vi "TLB Native Dynamic Events ver 0.26a.vi"() -> ()   [LabVIEW 2018] (continued)
              tunnel: [w1090 State_Type_Definitions,_for_0.26g_versions_and_later_2."True Stop" ("Enum")] -> w1083
              tunnel: [w1093 w1110] -> w1076
              tunnel: [State_Type_Definitions,_for_0.26g_versions_and_later_2."Idle" ("Enum") State_Type_Definitions,_for_0.26g_versions_and_later_2."Shutdown" ("Enum")] -> w1075
              tunnel: w1077 -> [w1084 _]
              tunnel: w1082 -> [w1089 w1107]
              tunnel: w1069 -> [w1088 _]
              frame "Start Task 1", Default {
                # ">> Is time up? >>"
                # "Determines if object is in range to pick up"
                # ">> Manual override >>"
                n408 = case shown="True" w1088 {
                  tunnel: [w1097 w1103] -> w1093
                  tunnel: w1089 -> [w1095 w1101]
                  frame False {
                    n409 = for {
                      tunnel: string[] ["Z STEPPER CAM HEIGHT", "READ STEPPER VALUES"] ("element") -> [w1098] mode=indexing
                      shift-right: [w1100] -> w1097
                      shift-left: w1095 -> [w1099]
                      n410 = Enqueue Element(queue=w1099, element=w1098) -> (queue out=w1100:refnum<queue>)  [unwired: 2 in, 2 out]
                    }
                  }
                  frame True {
                    n411 = for {
                      shift-right: [w1105] -> w1103
                      shift-left: w1101 -> [w1106]
                      tunnel: string[] ["SET TIMER 5", "", ""] -> [w1104] mode=indexing
                      n412 = Enqueue Element(queue=w1106, element=w1104) -> (queue out=w1105:refnum<queue>)  [unwired: 2 in, 2 out]
                    }
                  }
                }
                n413 = Or(x=w1088, y=w1084) -> (x .or. y?=w1091:bool)
                n414 = Select(t=State_Type_Definitions,_for_0.26g_versions_and_later_2."True Stop" ("Enum"), s=w1084, f=State_Type_Definitions,_for_0.26g_versions_and_later_2."Task 5D" ("Enum")) -> (s? t:f=w1086:T18)
                n415 = Select(t=w1086, s=w1091, f=State_Type_Definitions,_for_0.26g_versions_and_later_2."Task 5C" ("Enum")) -> (s? t:f=w1090:T18)
              }
              frame "Exit" {
                n416 = for {
                  shift-right: [w1113] -> w1110
                  shift-left: w1107 -> [w1114]
                  tunnel: string[] ["STOP", "RESET ENCODERS", "RESET YAW", "ARDUINO MODE 0"] -> [w1112] mode=indexing
                  n417 = Enqueue Element(queue=w1114, element=w1112) -> (queue out=w1113:refnum<queue>)  [unwired: 2 in, 2 out]
                }
              }
            }
          }
          frame 19 {
            # ">>> yStepper command>>>"
            n418 = Dequeue Element(queue=w1122, timeout in ms (-1)=w1121, error in (no error)=w1120) -> (element=w1119:T10)  [unwired: 3 out]
            n419 = case shown="\"Start Task 1\", Default" w1119 {
              tunnel: [w1134 State_Type_Definitions,_for_0.26g_versions_and_later_2."True Stop" ("Enum")] -> w1126
              tunnel: [w1137 w1154] -> w1125
              tunnel: [State_Type_Definitions,_for_0.26g_versions_and_later_2."Idle" ("Enum") State_Type_Definitions,_for_0.26g_versions_and_later_2."Shutdown" ("Enum")] -> w1127
              tunnel: w1123 -> [w1133 _]
              tunnel: w1124 -> [w1129 w1151]
              tunnel: w1117 -> [w1128 _]
              frame "Start Task 1", Default {
                # ">> T: Breaks out of state loop; F: Stays in loop>>"
                # ">> Manual override >>"
                # ">> Checks if time is up>>"
                # "Stays in Task 5D until the object is detected"
                # "T: Go back to idle, F: Continue with task\""
                # ">> Manual override >>"
                n420 = case shown="False" w1128 {
                  tunnel: [w1141 w1147] -> w1137
                  tunnel: w1129 -> [w1139 w1145]
                  frame False {
                    n421 = for {
                      tunnel: string[] ["START TIMER", "OPEN CLAW", ""] ("element") -> [w1142] mode=indexing
                      shift-right: [w1144] -> w1141
                      shift-left: w1139 -> [w1143]
                      n422 = Enqueue Element(queue=w1143, element=w1142) -> (queue out=w1144:refnum<queue>)  [unwired: 2 in, 2 out]
                    }
                  }
                  frame True {
                    n423 = for {
                      shift-right: [w1149] -> w1147
                      shift-left: w1145 -> [w1150]
                      tunnel: string[] ["CAM CLOSE", "", ""] -> [w1148] mode=indexing
                      n424 = Enqueue Element(queue=w1150, element=w1148) -> (queue out=w1149:refnum<queue>)  [unwired: 2 in, 2 out]
                    }
                  }
                }
                n425 = Or(x=w1128, y=w1133) -> (x .or. y?=w1135:bool)
                n426 = Select(t=State_Type_Definitions,_for_0.26g_versions_and_later_2."True Stop" ("Enum"), s=w1133, f=State_Type_Definitions,_for_0.26g_versions_and_later_2."True Stop" ("Enum")) -> (s? t:f=w1130:T18)
                n427 = Select(t=w1130, s=w1135, f=State_Type_Definitions,_for_0.26g_versions_and_later_2."Task 5D" ("Enum")) -> (s? t:f=w1134:T18)
              }
              frame "Exit" {
                n428 = for {
                  shift-right: [w1157] -> w1154
                  shift-left: w1151 -> [w1158]
                  tunnel: string[] ["STOP", "RESET ENCODERS", "RESET YAW", "ARDUINO MODE 0"] -> [w1156] mode=indexing
                  n429 = Enqueue Element(queue=w1158, element=w1156) -> (queue out=w1157:refnum<queue>)  [unwired: 2 in, 2 out]
                }
              }
            }
          }
          frame 20 {
            # ">>> yStepper command>>>"
            n430 = Dequeue Element(queue=w1172, timeout in ms (-1)=w1173, error in (no error)=w1174) -> (element=w1176:T10)  [unwired: 3 out]
            n431 = formula code="if (pos < 100)\ny = 41;\n\nelse if (pos >= 100 && pos <= 140)\ny = 30;\n\nelse if (pos >= 141 && pos <= 170)\ny = 25;\n\nelse if (pos >= 171 &&pos <= 180) \ny = 20;\n\nelse if (pos >= 181&& pos <= 200)\ny = 15;\n\nelse if (pos >= 201 && pos <= 230)\ny = 10;\n\nelse if (pos >= 231 && pos <= 320)\ny = 8;\n\nelse if (pos > 320)\ny = 0;"("pos"=w1164) -> ("y"=w1167:dbl)
            n432 = To Unsigned Byte Integer(number=w1167) -> (unsigned 8bit integer=w1162:u8)
            n433 = Equal?(x=w1163, y=w1162) -> (x = y?=w1161:bool)
            n434 = case shown="\"Start Task 1\", Default" w1176 {
              tunnel: [w1183 State_Type_Definitions,_for_0.26g_versions_and_later_2."True Stop" ("Enum")] -> w1170
              tunnel: [w1186 w1203] -> w1168
              tunnel: [State_Type_Definitions,_for_0.26g_versions_and_later_2."Idle" ("Enum") State_Type_Definitions,_for_0.26g_versions_and_later_2."Shutdown" ("Enum")] -> w1169
              tunnel: w1175 -> [w1182 _]
              tunnel: w1171 -> [w1178 w1200]
              tunnel: w1161 -> [w1177 _]
              frame "Start Task 1", Default {
                # ">> T: Breaks out of state loop; F: Stays in loop>>"
                # ">> Manual override >>"
                # ">> Checks if time is up>>"
                # "Stays in Task 5D until the object is detected"
                # "T: Go back to idle, F: Continue with task\""
                # ">> Manual override >>"
                n435 = case shown="False" w1177 {
                  tunnel: [w1190 w1196] -> w1186
                  tunnel: w1178 -> [w1188 w1194]
                  frame False {
                    n436 = for {
                      tunnel: string[] ["READ STEPPER VALUES", "Y STEPPER CONTROL", ""] ("element") -> [w1191] mode=indexing
                      shift-right: [w1193] -> w1190
                      shift-left: w1188 -> [w1192]
                      n437 = Enqueue Element(queue=w1192, element=w1191) -> (queue out=w1193:refnum<queue>)  [unwired: 2 in, 2 out]
                    }
                  }
                  frame True {
                    n438 = for {
                      shift-right: [w1198] -> w1196
                      shift-left: w1194 -> [w1199]
                      tunnel: string[] ["CAM CLOSE", "DISPOSE BUFFERS", ""] -> [w1197] mode=indexing
                      n439 = Enqueue Element(queue=w1199, element=w1197) -> (queue out=w1198:refnum<queue>)  [unwired: 2 in, 2 out]
                    }
                  }
                }
                n440 = Or(x=w1177, y=w1182) -> (x .or. y?=w1184:bool)
                n441 = Select(t=State_Type_Definitions,_for_0.26g_versions_and_later_2."True Stop" ("Enum"), s=w1182, f=State_Type_Definitions,_for_0.26g_versions_and_later_2."Task 5F: ARM GRAB HEIGHT" ("Enum")) -> (s? t:f=w1179:T18)
                n442 = Select(t=w1179, s=w1184, f=State_Type_Definitions,_for_0.26g_versions_and_later_2."Task 5E: POSITION ARM" ("Enum")) -> (s? t:f=w1183:T18)
              }
              frame "Exit" {
                n443 = for {
                  shift-right: [w1206] -> w1203
                  shift-left: w1200 -> [w1207]
                  tunnel: string[] ["STOP", "RESET ENCODERS", "RESET YAW", "ARDUINO MODE 0"] -> [w1205] mode=indexing
                  n444 = Enqueue Element(queue=w1207, element=w1205) -> (queue out=w1206:refnum<queue>)  [unwired: 2 in, 2 out]
                }
              }
            }
            n445 = Bundle By Name(cluster=w1166, "yStepper desired"=w1162) -> (w1165:T20)
          }
          frame 21 {
            # ">>> Motor control cluster >>>"
            # ">>> yStepper command>>>"
            # ">> Manual override >>"
            n446 = Dequeue Element(queue=w1218, timeout in ms (-1)=w1217, error in (no error)=w1219) -> (element=w1216:T10)  [unwired: 3 out]
            n447 = Equal?(x=w1215, y=u8 1) -> (x = y?=w1213:bool)
            n448 = case shown="\"Start Task 1\", Default" w1216 {
              tunnel: [w1229 State_Type_Definitions,_for_0.26g_versions_and_later_2."True Stop" ("Enum")] -> w1220
              tunnel: [w1232 w1249] -> w1221
              tunnel: [State_Type_Definitions,_for_0.26g_versions_and_later_2."Idle" ("Enum") State_Type_Definitions,_for_0.26g_versions_and_later_2."Shutdown" ("Enum")] -> w1222
              tunnel: w1213 -> [w1228 _]
              tunnel: w1212 -> [w1227 _]
              tunnel: w1211 -> [w1223 w1246]
              frame "Start Task 1", Default {
                # "Stays in Task 5F until stepper reaches desired \nheight"
                # "T: Go back to idle, F: Continue with task\""
                # ">> Manual override >>"
                n449 = case shown="True" w1228 {
                  tunnel: [w1236 w1242] -> w1232
                  tunnel: w1223 -> [w1234 w1240]
                  frame False {
                    n450 = for {
                      tunnel: string[] ["Z STEPPER GRAB HEIGHT", "READ STEPPER VALUES"] ("element") -> [w1237] mode=indexing
                      shift-right: [w1239] -> w1236
                      shift-left: w1234 -> [w1238]
                      n451 = Enqueue Element(queue=w1238, element=w1237) -> (queue out=w1239:refnum<queue>)  [unwired: 2 in, 2 out]
                    }
                  }
                  frame True {
                    n452 = for {
                      shift-right: [w1244] -> w1242
                      shift-left: w1240 -> [w1245]
                      tunnel: string[] ["SET TIMER 5", "CLOSE CLAW", ""] -> [w1243] mode=indexing
                      n453 = Enqueue Element(queue=w1245, element=w1243) -> (queue out=w1244:refnum<queue>)  [unwired: 2 in, 2 out]
                    }
                  }
                }
                n454 = Or(x=w1228, y=w1227) -> (x .or. y?=w1230:bool)
                n455 = Select(t=State_Type_Definitions,_for_0.26g_versions_and_later_2."True Stop" ("Enum"), s=w1227, f=State_Type_Definitions,_for_0.26g_versions_and_later_2."Task 5G: CLOSE CLAW" ("Enum")) -> (s? t:f=w1224:T18)
                n456 = Select(t=w1224, s=w1230, f=State_Type_Definitions,_for_0.26g_versions_and_later_2."Task 5F: ARM GRAB HEIGHT" ("Enum")) -> (s? t:f=w1229:T18)
              }
              frame "Exit" {
                n457 = for {
                  shift-right: [w1252] -> w1249
                  shift-left: w1246 -> [w1253]
                  tunnel: string[] ["STOP", "RESET ENCODERS", "RESET YAW", "ARDUINO MODE 0"] -> [w1251] mode=indexing
                  n458 = Enqueue Element(queue=w1253, element=w1251) -> (queue out=w1252:refnum<queue>)  [unwired: 2 in, 2 out]
                }
              }
            }
          }
          frame 22 {
            # ">>> yStepper command>>>"
            # ">> Manual override >>"
            n459 = Dequeue Element(queue=w1264, timeout in ms (-1)=w1263, error in (no error)=w1262) -> (element=w1261:T10)  [unwired: 3 out]
            n460 = case shown="\"Start Task 1\", Default" w1261 {
              tunnel: [w1273 State_Type_Definitions,_for_0.26g_versions_and_later_2."True Stop" ("Enum")] -> w1266
              tunnel: [w1276 w1293] -> w1259
              tunnel: [State_Type_Definitions,_for_0.26g_versions_and_later_2."Idle" ("Enum") State_Type_Definitions,_for_0.26g_versions_and_later_2."Shutdown" ("Enum")] -> w1258
              tunnel: w1260 -> [w1267 _]
              tunnel: w1265 -> [w1272 w1290]
              tunnel: w1256 -> [w1271 _]
              frame "Start Task 1", Default {
                # ">> Is time up? >>"
                # "Determines if object is in range to pick up"
                # ">> Manual override >>"
                n461 = case shown="True" w1271 {
                  tunnel: [w1280 w1286] -> w1276
                  tunnel: w1272 -> [w1278 w1284]
                  frame False {
                    n462 = for {
                      tunnel: string[] ["CLOSE CLAW", "START TIMER"] ("element") -> [w1281] mode=indexing
                      shift-right: [w1283] -> w1280
                      shift-left: w1278 -> [w1282]
                      n463 = Enqueue Element(queue=w1282, element=w1281) -> (queue out=w1283:refnum<queue>)  [unwired: 2 in, 2 out]
                    }
                  }
                  frame True {
                    n464 = for {
                      shift-right: [w1288] -> w1286
                      shift-left: w1284 -> [w1289]
                      tunnel: string[] ["READ STEPPER VALUES", "", ""] -> [w1287] mode=indexing
                      n465 = Enqueue Element(queue=w1289, element=w1287) -> (queue out=w1288:refnum<queue>)  [unwired: 2 in, 2 out]
                    }
                  }
                }
                n466 = Or(x=w1271, y=w1267) -> (x .or. y?=w1274:bool)
                n467 = Select(t=State_Type_Definitions,_for_0.26g_versions_and_later_2."True Stop" ("Enum"), s=w1267, f=State_Type_Definitions,_for_0.26g_versions_and_later_2."Task 5H: RAISE ARM" ("Enum")) -> (s? t:f=w1269:T18)
                n468 = Select(t=w1269, s=w1274, f=State_Type_Definitions,_for_0.26g_versions_and_later_2."Task 5G: CLOSE CLAW" ("Enum")) -> (s? t:f=w1273:T18)
              }
              frame "Exit" {
                n469 = for {
                  shift-right: [w1296] -> w1293
                  shift-left: w1290 -> [w1297]
                  tunnel: string[] ["STOP", "RESET ENCODERS", "RESET YAW", "ARDUINO MODE 0"] -> [w1295] mode=indexing
                  n470 = Enqueue Element(queue=w1297, element=w1295) -> (queue out=w1296:refnum<queue>)  [unwired: 2 in, 2 out]
                }
              }
            }
          }
          frame 23 {
            # ">>> yStepper command>>>"
            # ">> Manual override >>"
            n471 = Dequeue Element(queue=w1308, timeout in ms (-1)=w1307, error in (no error)=w1309) -> (element=w1306:T10)  [unwired: 3 out]
            n472 = Equal?(x=w1305, y=u8 60) -> (x = y?=w1303:bool)
            n473 = case shown="\"Start Task 1\", Default" w1306 {
              tunnel: [w1319 State_Type_Definitions,_for_0.26g_versions_and_later_2."True Stop" ("Enum")] -> w1310
              tunnel: [w1322 w1339] -> w1311
              tunnel: [State_Type_Definitions,_for_0.26g_versions_and_later_2."Idle" ("Enum") State_Type_Definitions,_for_0.26g_versions_and_later_2."Shutdown" ("Enum")] -> w1312
              tunnel: w1303 -> [w1318 _]
              tunnel: w1302 -> [w1317 _]
              tunnel: w1301 -> [w1313 w1336]
              frame "Start Task 1", Default {
                # "Stays in Task 5_A until stepper reaches desired \nheight"
                # "T: Go back to idle, F: Continue with task\""
                # ">> Manual override >>"
                n474 = case shown="False" w1318 {
                  tunnel: [w1326 w1332] -> w1322
                  tunnel: w1313 -> [w1324 w1330]
                  frame False {
                    n475 = for {
                      tunnel: string[] ["Z STEPPER CAM HEIGHT", "READ STEPPER VALUES"] ("element") -> [w1327] mode=indexing
                      shift-right: [w1329] -> w1326
                      shift-left: w1324 -> [w1328]
                      n476 = Enqueue Element(queue=w1328, element=w1327) -> (queue out=w1329:refnum<queue>)  [unwired: 2 in, 2 out]
                    }
                  }
                  frame True {
                    n477 = for {
                      shift-right: [w1334] -> w1332
                      shift-left: w1330 -> [w1335]
                      tunnel: string[] ["ARDUINO - ULTRASONIC", "READ ULTRASONIC", ""] -> [w1333] mode=indexing
                      n478 = Enqueue Element(queue=w1335, element=w1333) -> (queue out=w1334:refnum<queue>)  [unwired: 2 in, 2 out]
                    }
                  }
                }
                n479 = Or(x=w1318, y=w1317) -> (x .or. y?=w1320:bool)
                n480 = Select(t=State_Type_Definitions,_for_0.26g_versions_and_later_2."True Stop" ("Enum"), s=w1317, f=State_Type_Definitions,_for_0.26g_versions_and_later_2."True Stop" ("Enum")) -> (s? t:f=w1314:T18)
                n481 = Select(t=w1314, s=w1320, f=State_Type_Definitions,_for_0.26g_versions_and_later_2."Task 5H: RAISE ARM" ("Enum")) -> (s? t:f=w1319:T18)
              }
              frame "Exit" {
                n482 = for {
                  shift-right: [w1342] -> w1339
                  shift-left: w1336 -> [w1343]
                  tunnel: string[] ["STOP", "RESET ENCODERS", "RESET YAW", "ARDUINO MODE 0"] -> [w1341] mode=indexing
                  n483 = Enqueue Element(queue=w1343, element=w1341) -> (queue out=w1342:refnum<queue>)  [unwired: 2 in, 2 out]
                }
              }
            }
          }
          frame 24 {
            # ">>> yStepper command>>>"
            n484 = Dequeue Element(queue=w1353, timeout in ms (-1)=w1352, error in (no error)=w1351) -> (element=w1358:T10)  [unwired: 3 out]
            n485 = Equal?(x=w1349, y=u8 60) -> (x = y?=w1348:bool)
            n486 = case shown="\"Start Task 1\", Default" w1358 {
              tunnel: [w1365 State_Type_Definitions,_for_0.26g_versions_and_later_2."True Stop" ("Enum")] -> w1356
              tunnel: [w1364 w1382] -> w1355
              tunnel: [State_Type_Definitions,_for_0.26g_versions_and_later_2."Idle" ("Enum") State_Type_Definitions,_for_0.26g_versions_and_later_2."Shutdown" ("Enum")] -> w1357
              tunnel: w1354 -> [w1360 _]
              tunnel: w1350 -> [w1362 _]
              tunnel: w1348 -> [w1359 _]
              frame "Start Task 1", Default {
                n487 = case shown="False" w1359 {
                  tunnel: [w1370 w1376] -> w1364
                  tunnel: w1362 -> [w1368 w1374]
                  frame False {
                    n488 = for {
                      tunnel: string[] ["Z STEPPER CAM HEIGHT", "READ STEPPER VALUES"] ("element") -> [w1371] mode=indexing
                      shift-right: [w1373] -> w1370
                      shift-left: w1368 -> [w1372]
                      n489 = Enqueue Element(queue=w1372, element=w1371) -> (queue out=w1373:refnum<queue>)  [unwired: 2 in, 2 out]
                    }
                  }
                  frame True {
                    n490 = for {
                      shift-right: [w1378] -> w1376
                      shift-left: w1374 -> [w1379]
                      tunnel: string[] ["CAM ACQ", "OPEN LOG CAM"] -> [w1377] mode=indexing
                      n491 = Enqueue Element(queue=w1379, element=w1377) -> (queue out=w1378:refnum<queue>)  [unwired: 2 in, 2 out]
                    }
                  }
                }
                n492 = Or(x=w1359, y=w1360) -> (x .or. y?=w1361:bool)
                n493 = Select(t=State_Type_Definitions,_for_0.26g_versions_and_later_2."Task 6_B" ("Enum"), s=w1361, f=State_Type_Definitions,_for_0.26g_versions_and_later_2."Task 6_A" ("Enum")) -> (s? t:f=w1365:T18)
              }
              frame "Exit" {
                n494 = for {
                  shift-right: [w1385] -> w1382
                  shift-left: _ -> [w1386]
                  tunnel: string[] ["STOP", "RESET ENCODERS", "RESET YAW", "ARDUINO MODE 0"] -> [w1384] mode=indexing
                  n495 = Enqueue Element(queue=w1386, element=w1384) -> (queue out=w1385:refnum<queue>)  [unwired: 2 in, 2 out]
                }
              }
            }
          }
          frame 25 {
            # ">>> yStepper command>>>"
            n496 = Dequeue Element(queue=w1398, timeout in ms (-1)=w1396, error in (no error)=w1397) -> (element=w1395:T10)  [unwired: 3 out]
            n497 = case shown="\"Start Task 1\", Default" w1395 {
              tunnel: [w1405 State_Type_Definitions,_for_0.26g_versions_and_later_2."True Stop" ("Enum")] -> w1391
              tunnel: [w1404 w1423] -> w1399
              tunnel: [State_Type_Definitions,_for_0.26g_versions_and_later_2."Idle" ("Enum") State_Type_Definitions,_for_0.26g_versions_and_later_2."Shutdown" ("Enum")] -> w1392
              tunnel: w1394 -> [w1400 _]
              tunnel: w1393 -> [w1402 _]
              tunnel: w1390 -> [w1401 w1420]
              frame "Start Task 1", Default {
                # ">> Manual override >>"
                n498 = case shown="False" w1402 {
                  tunnel: [w1410 w1416] -> w1404
                  tunnel: w1401 -> [w1409 w1414]
                  frame False {
                    n499 = for {
                      shift-right: [w1413] -> w1410
                      shift-left: w1409 -> [w1412]
                      tunnel: string[] ["CAM ACQ", "PROCESS IMAGE", "OPEN CLAW"] -> [w1411] mode=indexing
                      n500 = Enqueue Element(queue=w1412, element=w1411) -> (queue out=w1413:refnum<queue>)  [unwired: 2 in, 2 out]
                    }
                  }
                  frame True {
                    n501 = for {
                      shift-right: [w1418] -> w1416
                      shift-left: w1414 -> [w1419]
                      tunnel: string[] ["CAM ACQ", "PROCESS IMAGE", "CLOSE CLAW"] -> [w1417] mode=indexing
                      n502 = Enqueue Element(queue=w1419, element=w1417) -> (queue out=w1418:refnum<queue>)  [unwired: 2 in, 2 out]
                    }
                  }
                }
                n503 = Select(t=State_Type_Definitions,_for_0.26g_versions_and_later_2."True Stop" ("Enum"), s=w1400, f=State_Type_Definitions,_for_0.26g_versions_and_later_2."Task 6_B" ("Enum")) -> (s? t:f=w1405:T18)
              }
              frame "Exit" {
                # ">> State after true stop >>"
                # ">> Goes to true stop >>"
                n504 = for {
                  shift-right: [w1426] -> w1423
                  shift-left: w1420 -> [w1427]
                  tunnel: string[] ["STOP", "RESET ENCODERS", "RESET YAW", ""] -> [w1425] mode=indexing
                  n505 = Enqueue Element(queue=w1427, element=w1425) -> (queue out=w1426:refnum<queue>)  [unwired: 2 in, 2 out]
                }
              }
            }
          }
          frame 26 {
          }
          frame 27 {
            # ">>> Motor control cluster >>>"
            # ">>> yStepper command>>>"
            # ">> Manual override >>"
            n506 = Dequeue Element(queue=w1444, timeout in ms (-1)=w1443, error in (no error)=w1445) -> (element=w1442:T10)  [unwired: 3 out]
            n507 = Equal?(x=w1441, y=u8 60) -> (x = y?=w1439:bool)
            n508 = case shown="\"Start Task 1\", Default" w1442 {
              tunnel: [w1455 State_Type_Definitions,_for_0.26g_versions_and_later_2."True Stop" ("Enum")] -> w1446
              tunnel: [w1458 w1475] -> w1447
              tunnel: [State_Type_Definitions,_for_0.26g_versions_and_later_2."Idle" ("Enum") State_Type_Definitions,_for_0.26g_versions_and_later_2."Shutdown" ("Enum")] -> w1448
              tunnel: w1439 -> [w1454 _]
              tunnel: w1438 -> [w1453 _]
              tunnel: w1437 -> [w1449 w1472]
              frame "Start Task 1", Default {
                # "Stays in Task 5_A until stepper reaches desired \nheight"
                # "T: Go back to idle, F: Continue with task\""
                # ">> Manual override >>"
                n509 = case shown="False" w1454 {
                  tunnel: [w1462 w1468] -> w1458
                  tunnel: w1449 -> [w1460 w1466]
                  frame False {
                    n510 = for {
                      tunnel: string[] ["Z STEPPER CAM HEIGHT", "READ STEPPER VALUES"] ("element") -> [w1463] mode=indexing
                      shift-right: [w1465] -> w1462
                      shift-left: w1460 -> [w1464]
                      n511 = Enqueue Element(queue=w1464, element=w1463) -> (queue out=w1465:refnum<queue>)  [unwired: 2 in, 2 out]
                    }
                  }
                  frame True {
                    n512 = for {
                      shift-right: [w1470] -> w1468
                      shift-left: w1466 -> [w1471]
                      tunnel: string[] ["ARDUINO - ULTRASONIC", "READ ULTRASONIC", ""] -> [w1469] mode=indexing
                      n513 = Enqueue Element(queue=w1471, element=w1469) -> (queue out=w1470:refnum<queue>)  [unwired: 2 in, 2 out]
                    }
                  }
                }
                n514 = Or(x=w1454, y=w1453) -> (x .or. y?=w1456:bool)
                n515 = Select(t=State_Type_Definitions,_for_0.26g_versions_and_later_2."True Stop" ("Enum"), s=w1453, f=State_Type_Definitions,_for_0.26g_versions_and_later_2."Task 8B: MOVE TO BOX" ("Enum")) -> (s? t:f=w1450:T18)
                n516 = Select(t=w1450, s=w1456, f=State_Type_Definitions,_for_0.26g_versions_and_later_2."Task 8A: RAISE ARM" ("Enum")) -> (s? t:f=w1455:T18)
              }
              frame "Exit" {
                n517 = for {
                  shift-right: [w1478] -> w1475
                  shift-left: w1472 -> [w1479]
                  tunnel: string[] ["STOP", "RESET ENCODERS", "RESET YAW", "ARDUINO MODE 0"] -> [w1477] mode=indexing
                  n518 = Enqueue Element(queue=w1479, element=w1477) -> (queue out=w1478:refnum<queue>)  [unwired: 2 in, 2 out]
                }
              }
            }
          }
          frame 28 {
            w1487 = u8 15 ("y")
            # ">>> yStepper command>>>"
            n519 = Less?(x=w1484, y=w1487) -> (x < y?=w1485:bool)
            n520 = Dequeue Element(queue=w1491, timeout in ms (-1)=w1490, error in (no error)=w1492) -> (element=w1489:T10)  [unwired: 3 out]
            n521 = Less?(x=w1483, y=w1487) -> (x < y?=w1486:bool)
            n522 = And(x=w1486, y=w1485) -> (x .and. y?=w1482:bool)
            n523 = case shown="\"Start Task 1\", Default" w1489 {
              tunnel: [w1504 State_Type_Definitions,_for_0.26g_versions_and_later_2."True Stop" ("Enum")] -> w1494
              tunnel: [w1507 w1524] -> w1493
              tunnel: [State_Type_Definitions,_for_0.26g_versions_and_later_2."Idle" ("Enum") State_Type_Definitions,_for_0.26g_versions_and_later_2."Shutdown" ("Enum")] -> w1495
              tunnel: w1497 -> [w1503 _]
              tunnel: w1496 -> [w1499 w1521]
              tunnel: w1482 -> [w1498 _]
              frame "Start Task 1", Default {
                # "Stays in Task 5_B to capture image over 5 seconds"
                # "T: Go back to idle, F: Continue with task\""
                # ">> Manual override >>"
                n524 = case shown="True" w1498 {
                  tunnel: [w1511 w1517] -> w1507
                  tunnel: w1499 -> [w1509 w1515]
                  frame False {
                    n525 = for {
                      tunnel: string[] ["FORWARD", "READ ULTRASONIC", "READ NAVX"] ("element") -> [w1512] mode=indexing
                      shift-right: [w1514] -> w1511
                      shift-left: w1509 -> [w1513]
                      n526 = Enqueue Element(queue=w1513, element=w1512) -> (queue out=w1514:refnum<queue>)  [unwired: 2 in, 2 out]
                    }
                  }
                  frame True {
                    n527 = for {
                      shift-right: [w1519] -> w1517
                      shift-left: w1515 -> [w1520]
                      tunnel: string[] ["STOP", "RESET ENCODERS", "OPEN LOG CAM", "SET TIMER 2", "OPEN IMAQ REF"] -> [w1518] mode=indexing
                      n528 = Enqueue Element(queue=w1520, element=w1518) -> (queue out=w1519:refnum<queue>)  [unwired: 2 in, 2 out]
                    }
                  }
                }
                n529 = Or(x=w1498, y=w1503) -> (x .or. y?=w1505:bool)
                n530 = Select(t=State_Type_Definitions,_for_0.26g_versions_and_later_2."True Stop" ("Enum"), s=w1503, f=State_Type_Definitions,_for_0.26g_versions_and_later_2."Task 8C: CAM BURST" ("Enum")) -> (s? t:f=w1500:T18)
                n531 = Select(t=w1500, s=w1505, f=State_Type_Definitions,_for_0.26g_versions_and_later_2."Task 8B: MOVE TO BOX" ("Enum")) -> (s? t:f=w1504:T18)
              }
              frame "Exit" {
                n532 = for {
                  shift-right: [w1527] -> w1524
                  shift-left: w1521 -> [w1528]
                  tunnel: string[] ["STOP", "RESET ENCODERS", "RESET YAW", "ARDUINO MODE 0"] -> [w1526] mode=indexing
                  n533 = Enqueue Element(queue=w1528, element=w1526) -> (queue out=w1527:refnum<queue>)  [unwired: 2 in, 2 out]
                }
              }
            }
          }
          frame 29 {
            # ">>> Motor control cluster >>>"
            # ">>> yStepper command>>>"
            # ">> Manual override >>"
            n534 = Dequeue Element(queue=w1539, timeout in ms (-1)=w1538, error in (no error)=w1537) -> (element=w1536:T10)  [unwired: 3 out]
            n535 = case shown="\"Start Task 1\", Default" w1536 {
              tunnel: [w1548 State_Type_Definitions,_for_0.26g_versions_and_later_2."True Stop" ("Enum")] -> w1541
              tunnel: [w1551 w1568] -> w1534
              tunnel: [State_Type_Definitions,_for_0.26g_versions_and_later_2."Idle" ("Enum") State_Type_Definitions,_for_0.26g_versions_and_later_2."Shutdown" ("Enum")] -> w1533
              tunnel: w1535 -> [w1542 _]
              tunnel: w1540 -> [w1547 w1565]
              tunnel: w1531 -> [w1546 _]
              frame "Start Task 1", Default {
                # ">> Is time up? >>"
                # "Determines if object is in range to pick up"
                # ">> Manual override >>"
                n536 = case shown="True" w1546 {
                  tunnel: [w1555 w1561] -> w1551
                  tunnel: w1547 -> [w1553 w1559]
                  frame False {
                    n537 = for {
                      tunnel: string[] ["CAM ACQ", "START TIMER"] ("element") -> [w1556] mode=indexing
                      shift-right: [w1558] -> w1555
                      shift-left: w1553 -> [w1557]
                      n538 = Enqueue Element(queue=w1557, element=w1556) -> (queue out=w1558:refnum<queue>)  [unwired: 2 in, 2 out]
                    }
                  }
                  frame True {
                    n539 = for {
                      shift-right: [w1563] -> w1561
                      shift-left: w1559 -> [w1564]
                      tunnel: string[] ["CAM CLOSE", "PROCESS IMAGE", "SET TIMER 5"] -> [w1562] mode=indexing
                      n540 = Enqueue Element(queue=w1564, element=w1562) -> (queue out=w1563:refnum<queue>)  [unwired: 2 in, 2 out]
                    }
                  }
                }
                n541 = Or(x=w1546, y=w1542) -> (x .or. y?=w1549:bool)
                n542 = Select(t=State_Type_Definitions,_for_0.26g_versions_and_later_2."True Stop" ("Enum"), s=w1542, f=State_Type_Definitions,_for_0.26g_versions_and_later_2."Task 8D: PROCESS IMAGE" ("Enum")) -> (s? t:f=w1544:T18)
                n543 = Select(t=w1544, s=w1549, f=State_Type_Definitions,_for_0.26g_versions_and_later_2."Task 8C: CAM BURST" ("Enum")) -> (s? t:f=w1548:T18)
              }
              frame "Exit" {
                n544 = for {
                  shift-right: [w1571] -> w1568
                  shift-left: w1565 -> [w1572]
                  tunnel: string[] ["STOP", "RESET ENCODERS", "RESET YAW", "ARDUINO MODE 0"] -> [w1570] mode=indexing
                  n545 = Enqueue Element(queue=w1572, element=w1570) -> (queue out=w1571:refnum<queue>)  [unwired: 2 in, 2 out]
                }
              }
            }
          }
          frame 30 {
            # ">>> yStepper command>>>"
            n546 = Dequeue Element(queue=w1580, timeout in ms (-1)=w1579, error in (no error)=w1578) -> (element=w1577:T10)  [unwired: 3 out]
            n547 = case shown="\"Start Task 1\", Default" w1577 {
              tunnel: [w1592 State_Type_Definitions,_for_0.26g_versions_and_later_2."True Stop" ("Enum")] -> w1584
              tunnel: [w1595 w1612] -> w1583
              tunnel: [State_Type_Definitions,_for_0.26g_versions_and_later_2."Idle" ("Enum") State_Type_Definitions,_for_0.26g_versions_and_later_2."Shutdown" ("Enum")] -> w1585
              tunnel: w1581 -> [w1591 _]
              tunnel: w1582 -> [w1587 w1609]
              tunnel: w1575 -> [w1586 _]
              frame "Start Task 1", Default {
                # ">> T: Breaks out of state loop; F: Stays in loop>>"
                # ">> Manual override >>"
                # ">> Checks if time is up>>"
                # "Stays in Task 5D until the object is detected"
                # "T: Go back to idle, F: Continue with task\""
                # ">> Manual override >>"
                n548 = case shown="True" w1586 {
                  tunnel: [w1599 w1605] -> w1595
                  tunnel: w1587 -> [w1597 w1603]
                  frame False {
                    n549 = for {
                      tunnel: string[] ["START TIMER", "PROCESS IMAGE", ""] ("element") -> [w1600] mode=indexing
                      shift-right: [w1602] -> w1599
                      shift-left: w1597 -> [w1601]
                      n550 = Enqueue Element(queue=w1601, element=w1600) -> (queue out=w1602:refnum<queue>)  [unwired: 2 in, 2 out]
                    }
                  }
                  frame True {
                    n551 = for {
                      shift-right: [w1607] -> w1605
                      shift-left: w1603 -> [w1608]
                      tunnel: string[] ["RESET ENCODERS", "", ""] -> [w1606] mode=indexing
                      n552 = Enqueue Element(queue=w1608, element=w1606) -> (queue out=w1607:refnum<queue>)  [unwired: 2 in, 2 out]
                    }
                  }
                }
                n553 = Or(x=w1586, y=w1591) -> (x .or. y?=w1593:bool)
                n554 = Select(t=State_Type_Definitions,_for_0.26g_versions_and_later_2."True Stop" ("Enum"), s=w1591, f=State_Type_Definitions,_for_0.26g_versions_and_later_2."Task 8E: ROBOT ADJUST" ("Enum")) -> (s? t:f=w1588:T18)
                n555 = Select(t=w1588, s=w1593, f=State_Type_Definitions,_for_0.26g_versions_and_later_2."Task 8D: PROCESS IMAGE" ("Enum")) -> (s? t:f=w1592:T18)
              }
              frame "Exit" {
                n556 = for {
                  shift-right: [w1615] -> w1612
                  shift-left: w1609 -> [w1616]
                  tunnel: string[] ["STOP", "RESET ENCODERS", "RESET YAW", "ARDUINO MODE 0"] -> [w1614] mode=indexing
                  n557 = Enqueue Element(queue=w1616, element=w1614) -> (queue out=w1615:refnum<queue>)  [unwired: 2 in, 2 out]
                }
              }
            }
          }
          frame 31 {
            # ">>> Motor control cluster >>>"
            # ">>> yStepper command>>>"
            n558 = Dequeue Element(queue=w1633, timeout in ms (-1)=w1632, error in (no error)=w1631) -> (element=w1630:T10)  [unwired: 3 out]
            n559 = Subtract(x=w1628, y=300.0) -> (x-y=w1626:dbl)
            n560 = formula code="if (error <= -61&&error > -300){\ndistance = -15;\nxSpeed = -30;\n}\n\nelse if (error <= -51 && error >= -60){\ndistance = -10;\nxSpeed = -30;\n}\n\nelse if (error >= -50 && error <= 50){\ndistance = 0;\nxSpeed = 0;\n}\n\nelse if (error >= 51 && error <= 80){\ndistance = 10;\nxSpeed = 30;\n}\n\nelse if (error >= 81 && error <= 100){\ndistance = 15;\nxSpeed = 30;\n}\n\nelse if (error >= 101 && error <= 120){\ndistance = 20;\nxSpeed = 30;\n}\n\nelse if (error >= 121 && error < 300){\ndistance = 25;\nxSpeed = 30;\n}\n\nelse{\ndistance = 0;\nxSpeed = 0;\n}"("error"=w1626) -> ("distance"=w1621:dbl, "xSpeed"=w1623:dbl)
            n561 = formula code="if (target > 0){\nif (current  >= target)\noutput = 1;\n\nelse if (current != target)\noutput = 0;\n}\n\nelse if (target == 0){\nif (current == target)\noutput = 1;\n\nelse if (current != target)\noutput = 0;\n}\n\nelse if (target < 0){\nif (current <= target)\noutput = 1;\n\nelse if (current != target)\noutput = 0;\n}\n\nelse if (current != target)\noutput = 0;"("target"=w1621, "current"=w1622) -> ("output"=w1620:dbl)
            n562 = Bundle By Name(cluster=w1625, "xSpeed"=w1623) -> (w1624:T19)
            n563 = Equal?(x=w1620, y=1.0) -> (x = y?=w1618:bool)
            n564 = case shown="\"Start Task 1\", Default" w1630 {
              tunnel: [w1645 State_Type_Definitions,_for_0.26g_versions_and_later_2."True Stop" ("Enum")] -> w1637
              tunnel: [w1648 w1665] -> w1636
              tunnel: [State_Type_Definitions,_for_0.26g_versions_and_later_2."Idle" ("Enum") State_Type_Definitions,_for_0.26g_versions_and_later_2."Shutdown" ("Enum")] -> w1638
              tunnel: w1634 -> [w1644 _]
              tunnel: w1635 -> [w1640 w1662]
              tunnel: w1618 -> [w1639 _]
              frame "Start Task 1", Default {
                # ">> T: Breaks out of state loop; F: Stays in loop>>"
                # ">> Manual override >>"
                # ">> Checks if time is up>>"
                # "Stays in Task 5D until the object is detected"
                # "T: Go back to idle, F: Continue with task\""
                # ">> Manual override >>"
                n565 = case shown="True" w1639 {
                  tunnel: [w1652 w1658] -> w1648
                  tunnel: w1640 -> [w1650 w1656]
                  frame False {
                    n566 = for {
                      tunnel: string[] ["X AXIS - SLOW", "READ ENCODERS", "READ NAVX"] ("element") -> [w1653] mode=indexing
                      shift-right: [w1655] -> w1652
                      shift-left: w1650 -> [w1654]
                      n567 = Enqueue Element(queue=w1654, element=w1653) -> (queue out=w1655:refnum<queue>)  [unwired: 2 in, 2 out]
                    }
                  }
                  frame True {
                    n568 = for {
                      shift-right: [w1660] -> w1658
                      shift-left: w1656 -> [w1661]
                      tunnel: string[] ["SET TIMER 2", "STOP", "READ STEPPER VALUES", ""] -> [w1659] mode=indexing
                      n569 = Enqueue Element(queue=w1661, element=w1659) -> (queue out=w1660:refnum<queue>)  [unwired: 2 in, 2 out]
                    }
                  }
                }
                n570 = Or(x=w1639, y=w1644) -> (x .or. y?=w1646:bool)
                n571 = Select(t=State_Type_Definitions,_for_0.26g_versions_and_later_2."True Stop" ("Enum"), s=w1644, f=State_Type_Definitions,_for_0.26g_versions_and_later_2."Task 8H: ARM ADJUST" ("Enum")) -> (s? t:f=w1641:T18)
                n572 = Select(t=w1641, s=w1646, f=State_Type_Definitions,_for_0.26g_versions_and_later_2."Task 8E: ROBOT ADJUST" ("Enum")) -> (s? t:f=w1645:T18)
              }
              frame "Exit" {
                n573 = for {
                  shift-right: [w1668] -> w1665
                  shift-left: w1662 -> [w1669]
                  tunnel: string[] ["STOP", "RESET ENCODERS", "RESET YAW", "ARDUINO MODE 0"] -> [w1667] mode=indexing
                  n574 = Enqueue Element(queue=w1669, element=w1667) -> (queue out=w1668:refnum<queue>)  [unwired: 2 in, 2 out]
                }
              }
            }
          }
          frame 32 {
            # ">>> Motor control cluster >>>"
            # ">>> yStepper command>>>"
            # ">> Manual override >>"
            n575 = Dequeue Element(queue=w1680, timeout in ms (-1)=w1679, error in (no error)=w1678) -> (element=w1677:T10)  [unwired: 3 out]
            n576 = case shown="\"Start Task 1\", Default" w1677 {
              tunnel: [w1689 State_Type_Definitions,_for_0.26g_versions_and_later_2."True Stop" ("Enum")] -> w1682
              tunnel: [w1692 w1709] -> w1675
              tunnel: [State_Type_Definitions,_for_0.26g_versions_and_later_2."Idle" ("Enum") State_Type_Definitions,_for_0.26g_versions_and_later_2."Shutdown" ("Enum")] -> w1674
              tunnel: w1676 -> [w1683 _]
              tunnel: w1681 -> [w1688 w1706]
              tunnel: w1672 -> [w1687 _]
              frame "Start Task 1", Default {
                # ">> Is time up? >>"
                # "Determines if object is in range to pick up"
                # ">> Manual override >>"
                n577 = case shown="False" w1687 {
                  tunnel: [w1696 w1702] -> w1692
                  tunnel: w1688 -> [w1694 w1700]
                  frame False {
                    n578 = for {
                      tunnel: string[] ["CAM ACQ", "START TIMER"] ("element") -> [w1697] mode=indexing
                      shift-right: [w1699] -> w1696
                      shift-left: w1694 -> [w1698]
                      n579 = Enqueue Element(queue=w1698, element=w1697) -> (queue out=w1699:refnum<queue>)  [unwired: 2 in, 2 out]
                    }
                  }
                  frame True {
                    n580 = for {
                      shift-right: [w1704] -> w1702
                      shift-left: w1700 -> [w1705]
                      tunnel: string[] ["CAM CLOSE", "PROCESS IMAGE", "SET TIMER 3"] -> [w1703] mode=indexing
                      n581 = Enqueue Element(queue=w1705, element=w1703) -> (queue out=w1704:refnum<queue>)  [unwired: 2 in, 2 out]
                    }
                  }
                }
                n582 = Or(x=w1687, y=w1683) -> (x .or. y?=w1690:bool)
                n583 = Select(t=State_Type_Definitions,_for_0.26g_versions_and_later_2."True Stop" ("Enum"), s=w1683, f=State_Type_Definitions,_for_0.26g_versions_and_later_2."Task 8G: PROCESS IMAGE 2" ("Enum")) -> (s? t:f=w1685:T18)
                n584 = Select(t=w1685, s=w1690, f=State_Type_Definitions,_for_0.26g_versions_and_later_2."Task 8F: CAM BURST 2" ("Enum")) -> (s? t:f=w1689:T18)
              }
              frame "Exit" {
                n585 = for {
                  shift-right: [w1712] -> w1709
                  shift-left: w1706 -> [w1713]
                  tunnel: string[] ["STOP", "RESET ENCODERS", "RESET YAW", "ARDUINO MODE 0"] -> [w1711] mode=indexing
                  n586 = Enqueue Element(queue=w1713, element=w1711) -> (queue out=w1712:refnum<queue>)  [unwired: 2 in, 2 out]
                }
              }
            }
          }
          frame 33 {
            # ">>> yStepper command>>>"
            n587 = Dequeue Element(queue=w1721, timeout in ms (-1)=w1720, error in (no error)=w1719) -> (element=w1718:T10)  [unwired: 3 out]
            n588 = case shown="\"Start Task 1\", Default" w1718 {
              tunnel: [w1733 State_Type_Definitions,_for_0.26g_versions_and_later_2."True Stop" ("Enum")] -> w1725
              tunnel: [w1736 w1753] -> w1724
              tunnel: [State_Type_Definitions,_for_0.26g_versions_and_later_2."Idle" ("Enum") State_Type_Definitions,_for_0.26g_versions_and_later_2."Shutdown" ("Enum")] -> w1726
              tunnel: w1722 -> [w1732 _]
              tunnel: w1723 -> [w1728 w1750]
              tunnel: w1716 -> [w1727 _]
              frame "Start Task 1", Default {
                # ">> T: Breaks out of state loop; F: Stays in loop>>"
                # ">> Manual override >>"
                # ">> Checks if time is up>>"
                # "Stays in Task 5D until the object is detected"
                # "T: Go back to idle, F: Continue with task\""
                # ">> Manual override >>"
                n589 = case shown="False" w1727 {
                  tunnel: [w1740 w1746] -> w1736
                  tunnel: w1728 -> [w1738 w1744]
                  frame False {
                    n590 = for {
                      tunnel: string[] ["START TIMER", "PROCESS IMAGE", ""] ("element") -> [w1741] mode=indexing
                      shift-right: [w1743] -> w1740
                      shift-left: w1738 -> [w1742]
                      n591 = Enqueue Element(queue=w1742, element=w1741) -> (queue out=w1743:refnum<queue>)  [unwired: 2 in, 2 out]
                    }
                  }
                  frame True {
                    n592 = for {
                      shift-right: [w1748] -> w1746
                      shift-left: w1744 -> [w1749]
                      tunnel: string[] ["READ STEPPER VALUES", "Y STEPPER CONTROL", ""] -> [w1747] mode=indexing
                      n593 = Enqueue Element(queue=w1749, element=w1747) -> (queue out=w1748:refnum<queue>)  [unwired: 2 in, 2 out]
                    }
                  }
                }
                n594 = Or(x=w1727, y=w1732) -> (x .or. y?=w1734:bool)
                n595 = Select(t=State_Type_Definitions,_for_0.26g_versions_and_later_2."True Stop" ("Enum"), s=w1732, f=State_Type_Definitions,_for_0.26g_versions_and_later_2."Task 8H: ARM ADJUST" ("Enum")) -> (s? t:f=w1729:T18)
                n596 = Select(t=w1729, s=w1734, f=State_Type_Definitions,_for_0.26g_versions_and_later_2."Task 8G: PROCESS IMAGE 2" ("Enum")) -> (s? t:f=w1733:T18)
              }
              frame "Exit" {
                n597 = for {
                  shift-right: [w1756] -> w1753
                  shift-left: w1750 -> [w1757]
                  tunnel: string[] ["STOP", "RESET ENCODERS", "RESET YAW", "ARDUINO MODE 0"] -> [w1755] mode=indexing
                  n598 = Enqueue Element(queue=w1757, element=w1755) -> (queue out=w1756:refnum<queue>)  [unwired: 2 in, 2 out]
                }
              }
            }
          }
          frame 34 {
            # ">>> yStepper command>>>"
            n599 = Dequeue Element(queue=w1771, timeout in ms (-1)=w1772, error in (no error)=w1773) -> (element=w1775:T10)  [unwired: 3 out]
            n600 = formula code="if (pos < 70)\ny = 43;\n\nelse if (pos >= 71 &&pos <= 80)\ny = 40;\n\nelse if (pos >= 81 && pos <= 90)\ny = 38;\n\nelse if (pos >= 91 &&pos <= 120)\ny = 35;\n\nelse if (pos >= 121 && pos <= 140)\ny = 30;\n\nelse if (pos >= 141 && pos <= 170)\ny = 26;\n\nelse if (pos >= 171 &&pos <= 220) \ny = 20;\n\nelse if (pos >= 221&& pos <= 240)\ny = 15;\n\nelse if (pos >= 241 && pos <= 250)\ny = 10;\n\nelse if (pos >= 251)\ny = 0;"("pos"=w1763) -> ("y"=w1766:dbl)
            n601 = To Unsigned Byte Integer(number=w1766) -> (unsigned 8bit integer=w1761:u8)
            n602 = Equal?(x=w1762, y=w1761) -> (x = y?=w1760:bool)
            n603 = case shown="\"Start Task 1\", Default" w1775 {
              tunnel: [w1782 State_Type_Definitions,_for_0.26g_versions_and_later_2."True Stop" ("Enum")] -> w1769
              tunnel: [w1785 w1802] -> w1767
              tunnel: [State_Type_Definitions,_for_0.26g_versions_and_later_2."Idle" ("Enum") State_Type_Definitions,_for_0.26g_versions_and_later_2."Shutdown" ("Enum")] -> w1768
              tunnel: w1774 -> [w1781 _]
              tunnel: w1770 -> [w1777 w1799]
              tunnel: w1760 -> [w1776 _]